vi "VP_RT_base.vi"() -> ()   [LabVIEW 2015] (continued)
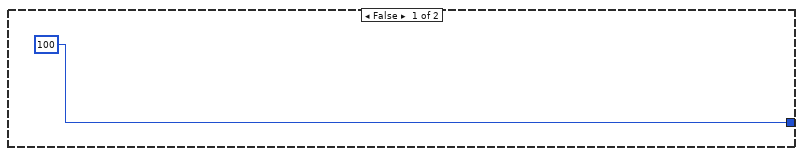
[diagram p2: hidden frame]
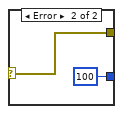
[diagram p3: hidden frame]
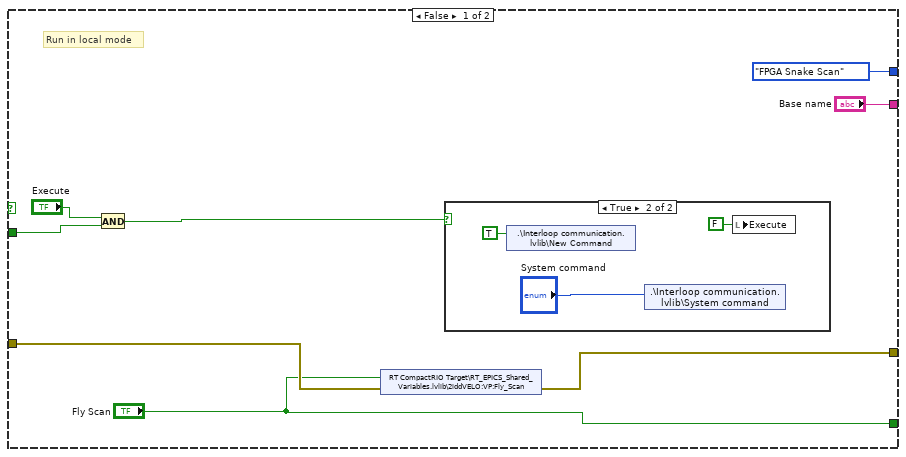
[diagram p4: hidden frame]
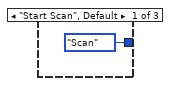
[diagram p7: hidden frame]
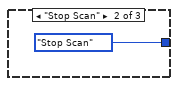
[diagram p8: hidden frame]
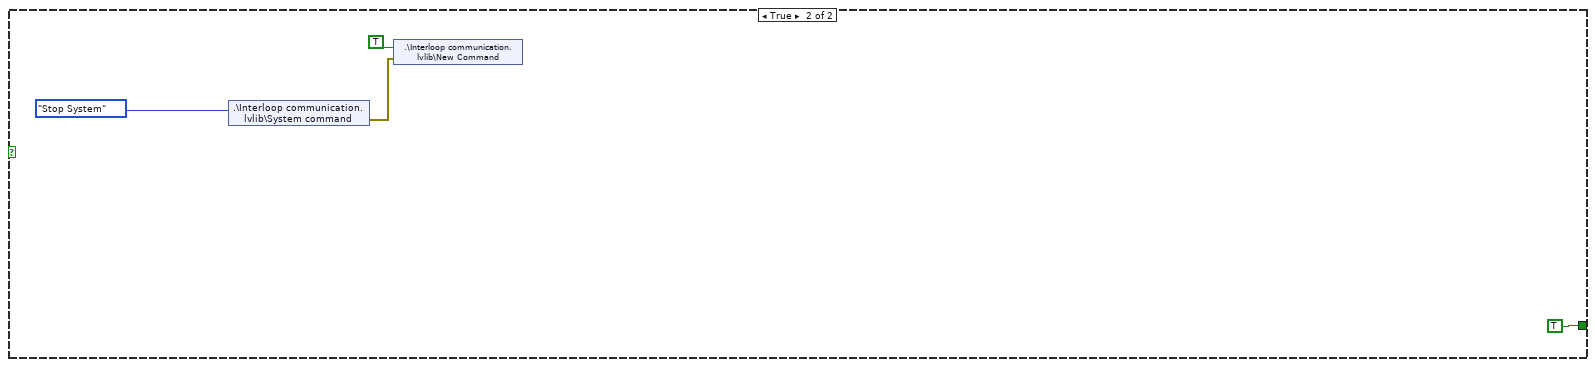
[diagram p9: hidden frame]
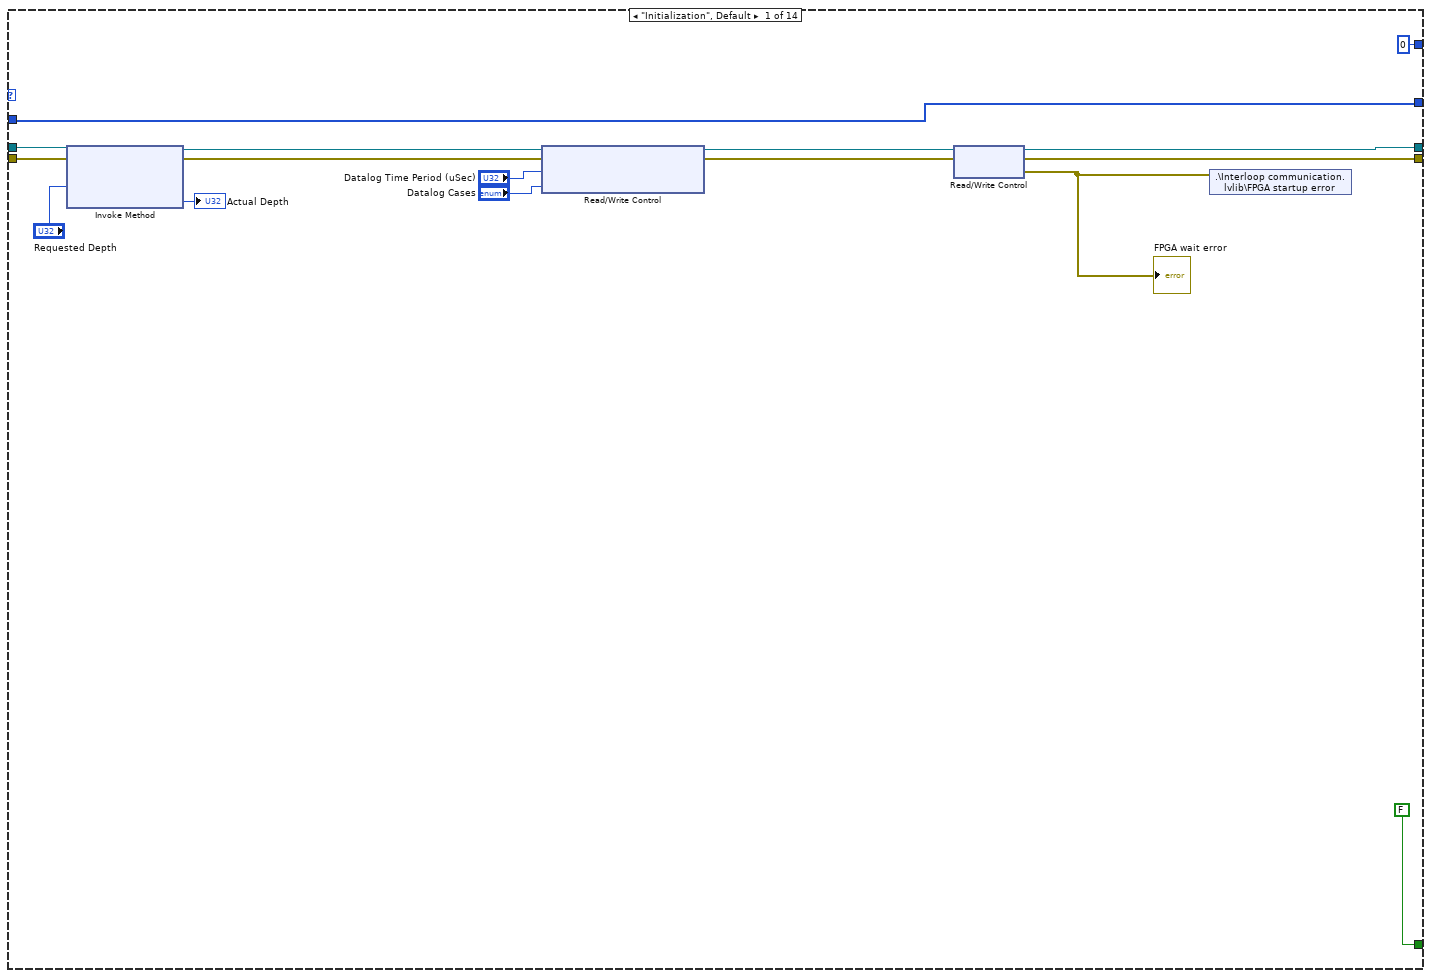
[diagram p10: hidden frame]
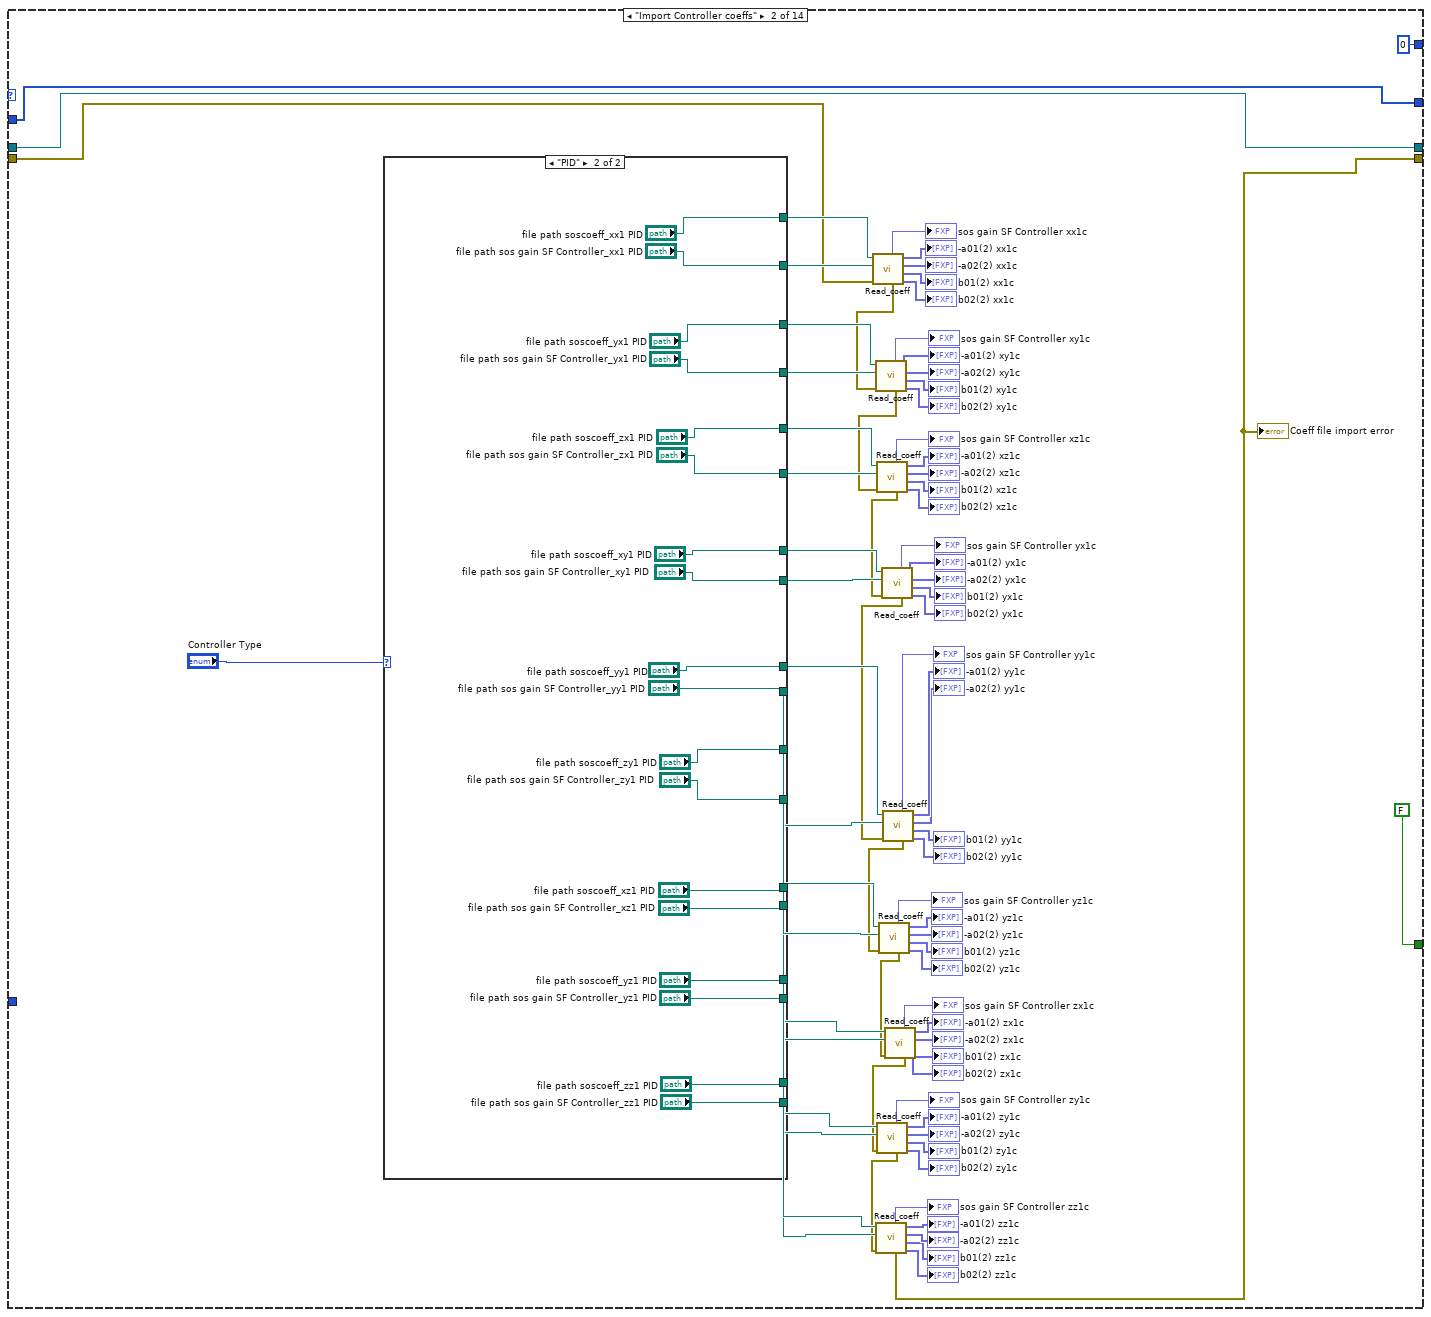
[diagram p11: hidden frame]
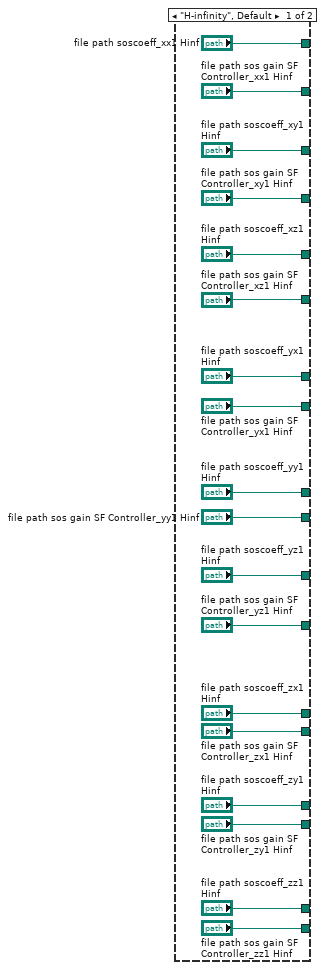
[diagram p12: hidden frame]
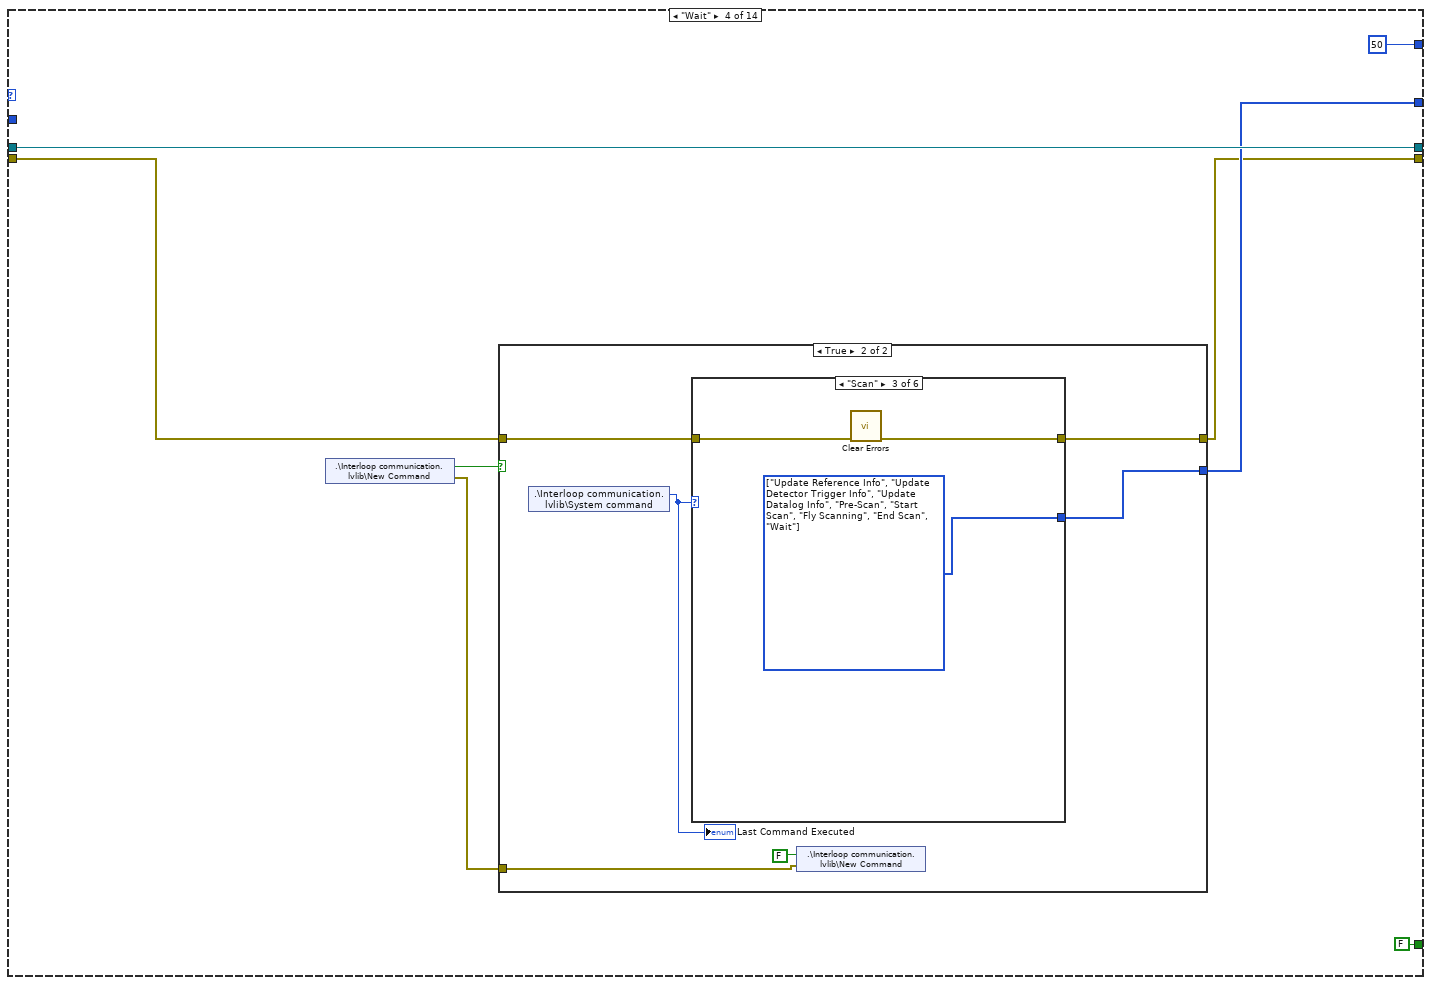
[diagram p13: hidden frame]
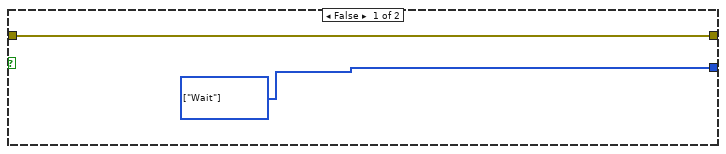
[diagram p14: hidden frame]
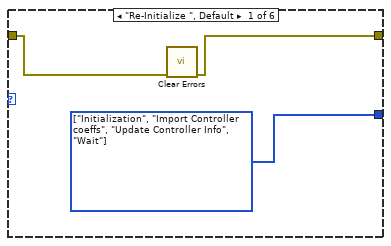
[diagram p15: hidden frame]
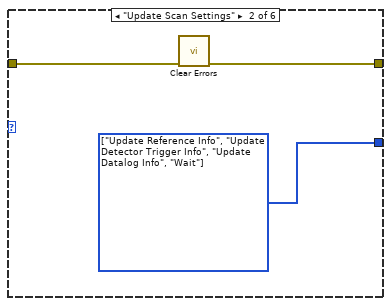
[diagram p16: hidden frame]
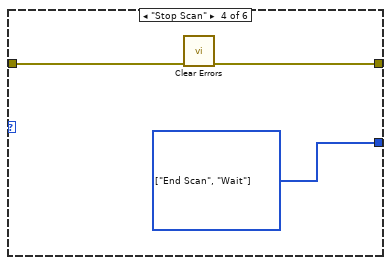
[diagram p17: hidden frame]
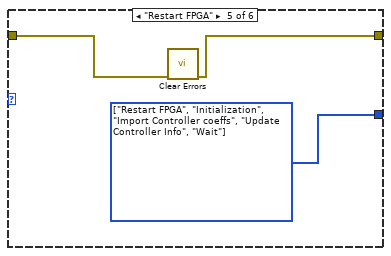
[diagram p18: hidden frame]
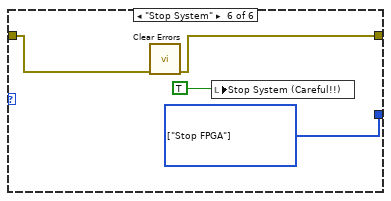
[diagram p19: hidden frame]
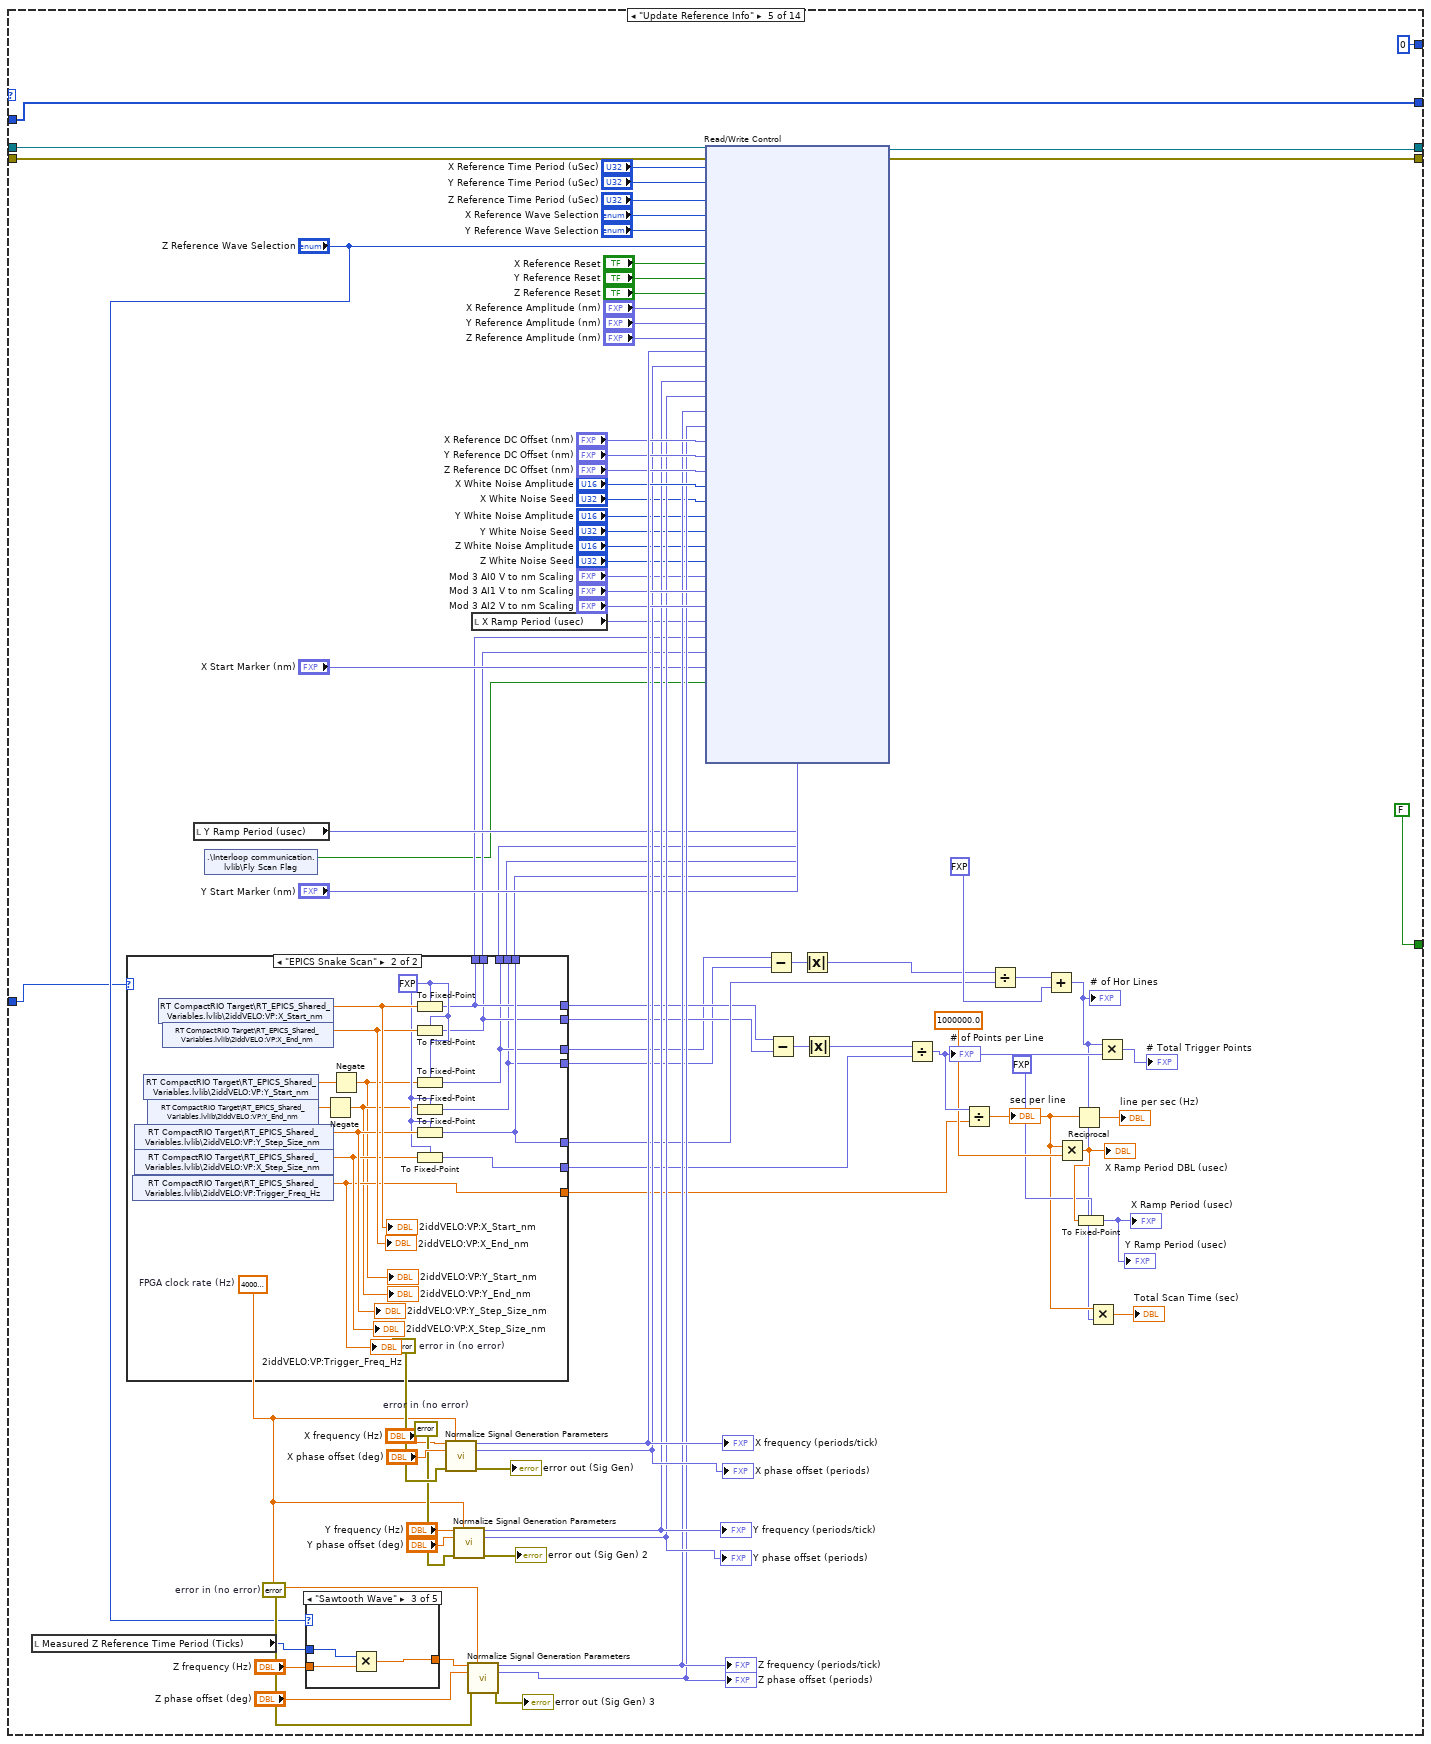
[diagram p20: hidden frame]
        n230 = case shown="False" w615 {
          tunnel: w614 -> [w668 w669]
          tunnel: [w666 w669] -> w613
          frame False {
            # "Either FIFO not empty or FPGA not \ndone running -- repeat scanning state"
            n231 = Insert Into Array(array=w668, index=0, new element=State_Enum."Fly Scanning" ("new element/subarray")) -> (w666:T11[])
          }
          frame True {
            # "FIFO empty, FPGA done running \n-- moving onto next state"
          }
        }
        n232 = Bundle("t0"=w662, w657, w658) -> (→"Reference and Actual positions":cluster{"t0":dbl, dbl, dbl[][]})  [unwired: 1 in]
        n233 = Array To Spreadsheet String(delimiter (Tab)=w634, array=w653, 3:w635) -> (spreadsheet string=w633:string)
        n234 = call "Convert to Dynamic Data"("Array"=w611) -> ("Dynamic Data Type"=w648:dynamicdata)  [unwired: 3 in]
        n235 = call "Convert to Dynamic Data2"("Array"=w610) -> ("Dynamic Data Type"=w642:dynamicdata)  [unwired: 3 in]
        n236 = call "Convert to Dynamic Data3"("Array"=w609) -> ("Dynamic Data Type"=w644:dynamicdata)  [unwired: 3 in]
        n237 = call "Convert to Dynamic Data4"("Array"=w608) -> ("Dynamic Data Type"=w643:dynamicdata)  [unwired: 3 in]
        n238 = call "Data_Write.vi"("error initialize"=w654, "Data"=w633, "Command List"=Data_Write_Control."Write") -> ("error out"=w632:errorcluster)  [unwired: 5 in, 1 out]
        n239 = To Double Precision Float(number=w611) -> (double precision float=w607:dbl[])
        n240 = To Double Precision Float(number=w610) -> (double precision float=w606:dbl[])
        n241 = To Double Precision Float(number=w609) -> (double precision float=w605:dbl[])
        n242 = To Double Precision Float(number=w608) -> (double precision float=w604:dbl[])
        n243 = call "Convert from Dynamic Data"("Dynamic Data Type"=w648) -> ("Array"=w649:dbl[])  [unwired: 3 in]
        n244 = call "Convert from Dynamic Data2"("Dynamic Data Type"=w642) -> ("Array"=w647:dbl[])  [unwired: 3 in]
        n245 = call "Convert from Dynamic Data3"("Dynamic Data Type"=w644) -> ("Array"=w646:dbl[])  [unwired: 3 in]
        n246 = call "Convert from Dynamic Data4"("Dynamic Data Type"=w643) -> ("Array"=w645:dbl[])  [unwired: 3 in]
        n247 = Bundle(w605, w604) -> (→"XY Graph 4":cluster{dbl[], dbl[]})  [unwired: 1 in]
        n248 = Bundle(w607, w606) -> (→"XY Graph 3":cluster{dbl[], dbl[]})  [unwired: 1 in]
        n249 = Bundle("Array"=w649, "Array"=w647) -> (→"XY Ref":cluster{"Array":dbl[], "Array":dbl[]})  [unwired: 1 in]
        n250 = Bundle("Array"=w646, "Array"=w645) -> (→"XY actual":cluster{"Array":dbl[], "Array":dbl[]})  [unwired: 1 in]
        n251 = Merge Errors(w638, w632) -> (w637:errorcluster)
      }
      frame "End Scan" {
        n252 = xnode "Invoke Method"("FPGA VI Reference In"=w675, "error in"=w673) -> ("FPGA VI Reference Out"=w674:refnum<k20>, "error out"=w672:errorcluster)
        n253 = xnode "Read/Write Control"("FPGA VI Reference In"=w674, "error in"=w672, "stop case"=TRUE ("New FPGA command")) -> ("FPGA VI Reference Out"=w678:refnum<k20>, "error out"=w677:errorcluster)
        n254 = shared-variable "RT CompactRIO Target\\RT_EPICS_Shared_Variables.lvlib\\2iddVELO:VP:Scanning"(FALSE ("2iddVELO:VP:Fly_Scanning")) -> ()  [unwired: 1 in, 1 out]
        n255 = call "Data_Write.vi"("error initialize"=w677, "Command List"=Data_Write_Control."Close") -> ("error out"=w671:errorcluster)  [unwired: 6 in, 1 out]
        n256 = case shown="No Error" w671 {
          tunnel: w671 -> [w689 w690]
          tunnel: [w688 w690] -> w681
          frame No Error {
            n257 = local read "Output filename"() -> (w685:string)
            n258 = local read "Output path"() -> (w686:path)
            n259 = Path To String(path=w686) -> (string=w684:string)
            n260 = shared-variable "RT CompactRIO Target\\RT_EPICS_Shared_Variables.lvlib\\2iddVELO:VP:Last_Filename"(w685, error in=w689) -> (error out=w687:errorcluster)
            n261 = shared-variable "RT CompactRIO Target\\RT_EPICS_Shared_Variables.lvlib\\2iddVELO:VP:cRIO_Dir"(w684, error in=w687) -> (error out=w688:errorcluster)
          }
          frame Error {
          }
        }
      }
      frame "Restart FPGA" {
        n262 = call <vilib>:"Clear Errors.vi"("error in (no error)"=w696) -> ("error out"=w697:errorcluster)  [unwired: 5 in, 1 out]
        n263 = xnode "Invoke Method"("FPGA VI Reference In"=w702, "error in"=w697) -> ("FPGA VI Reference Out"=w701:refnum<k20>, "error out"=w700:errorcluster)
        n264 = xnode "Read/Write Control"("FPGA VI Reference In"=w701, "error in"=w700, "stop case"=TRUE) -> ("FPGA VI Reference Out"=w695:refnum<k20>, "error out"=w694:errorcluster)
        n265 = xnode "Invoke Method"("FPGA VI Reference In"=w695, "error in"=w694) -> ("FPGA VI Reference Out"=w693:refnum<k20>, "error out"=w692:errorcluster)
      }
      frame "Stop FPGA" {
        w710 = T11[] [enum."Stop FPGA"] items=["Initialization", "Import Controller coeffs", "Update Controller Info", "Wait", "Update Reference Info", "Update Detector Trigger Info", "Update Datalog Info", "Check FPGA Status", "Pre-Scan", "Start Scan", "Step Scanning", "Fly Scanning", "End Scan", "Restart FPGA", "Stop FPGA"] ("Reduced Array of States")
        w709 = TRUE ("stop case")
        n266 = xnode "Invoke Method"("FPGA VI Reference In"=w717, "error in"=w716) -> ("FPGA VI Reference Out"=w715:refnum<k20>, "error out"=w714:errorcluster)
        n267 = xnode "Read/Write Control"("FPGA VI Reference In"=w715, "error in"=w714, "stop case"=w709, "New FPGA command"=w709, "FPGA command"=enum16{"Start Scan", "Shutdown"}."Shutdown") -> ("FPGA VI Reference Out"=w713:refnum<k20>, "error out"=w706:errorcluster)
        n268 = xnode "Invoke Method"("FPGA VI Reference In"=w713, "error in"=w706) -> ("FPGA VI Reference Out"=w707:refnum<k20>, "error out"=w705:errorcluster)
        n269 = xnode "Close FPGA VI Reference"("FPGA VI Reference In"=w707, "error in"=w705) -> ("error out"=w712:errorcluster)
      }
    }
    "Main Loop error" <- w105
    n270 = shared-variable ".\\Interloop communication.lvlib\\Main Loop Error"(w105) -> ()  [unwired: 1 in, 1 out]
    n271 = node-c288(w100) -> ()  [unwired: 1 out]
    n272 = call "State Control.vi"("Stop"=FALSE, "Array of States"=w107, "Error Input"=w105) -> ("Next State"=w97:T11, "Reduced Array of States"=w101:T11[])  [unwired: 5 in]
    "RT Main Loop State" <- w94
    "Main Loop Iterations" <- w103
    "Reduced Array of States" <- w102
  }
  n273 = while {
    tunnel: w2 -> [w726]
    tunnel: w1 -> [w725]
    i -> [w723]
    stop <- w724 stop-if-true
    # "Readback loop"
    n274 = local read "RT Main Loop State"() -> (w729:T11)
    n275 = Not Equal?(x=w729, y=State_Enum."Initialization") -> (x != y?=w727:bool)
    n276 = case shown="True" w727 {
      tunnel: w726 -> [_ w737]
      tunnel: w725 -> [_ w735]
      tunnel: [u32 100 ("milliseconds to wait") "Readback Loop time between iterations (ms)"] -> w722
      frame False {
      }
      frame True {
        w776 = 40000000.0  # FPGA Clock Rate (Hz)
        w795 = 40000000.0  # FPGA Clock Rate (Hz)
        w812 = 40000000.0  # FPGA Clock Rate (Hz)
        n277 = xnode "Read/Write Control"("FPGA VI Reference In"=w737, "error in"=w735) -> ("FPGA VI Reference Out"=w736:refnum<k20>, "error out"=w734:errorcluster, "FPGA state"=w733:T10, "Fly scan completed"=→"Fly Scan Complete":bool)
        "FPGA state" <- w733
        n278 = Format Into String(format string="%s", w733) -> (resulting string=w732:string)  [unwired: 2 in, 1 out]
        n279 = xnode "Read/Write Control"("FPGA VI Reference In"=w736, "error in"=w734) -> ("error out"=w743:errorcluster, "Measured Datalog Time Period (Ticks)"=w770:u32, "Measured Counter Time Period (Ticks)"=w775:u32, "Mod4/DIO0"=→"Mod4/DIO0":bool, "Mod4/DIO1"=→"Mod4/DIO1":bool, "Mod4/DIO2"=→"Mod4/DIO2":bool, "Mod4/DIO3"=→"Mod4/DIO3":bool, "Mod5/DIO0"=→"Mod5/DIO0":bool, "Mod5/DIO1"=→"Mod5/DIO1":bool, "Mod5/DIO2"=→"Mod5/DIO2":bool, "Mod5/DIO3"=→"Mod5/DIO3":bool, "Mod6/DIO0"=→"Mod6/DIO0":bool, "Mod6/DIO1"=→"Mod6/DIO1":bool, "Mod6/DIO2"=→"Mod6/DIO2":bool, "Mod6/DIO3"=→"Mod6/DIO3":bool, "32 bit Count Optics X"=→"32 bit Count Optics X":i32, "32 bit Count Optics  Y"=→"32 bit Count Optics  Y":i32, "32 bit Count Optics  Z"=→"32 bit Count Optics  Z":i32, "32 bit Count Sample X"=→"32 bit Count Sample X":i32, "32 bit Count Sample  Y"=→"32 bit Count Sample  Y":i32, "32 bit Count Sample  Z"=→"32 bit Count Sample  Z":i32, "Optics X Stage Displacement (nm)"=→"Optics X Stage Displacement (nm)":fxp<+/-,58,25>, "Optics Y Stage Displacement (nm)"=→"Optics Y Stage Displacement (nm)":fxp<+/-,58,25>, "Optics Z Stage Displacement (nm)"=→"Optics Z Stage Displacement (nm)":fxp<+/-,58,25>, "Sample X Stage Displacement (nm)"=→"Sample X Stage Displacement (nm)":fxp<+/-,58,25>, "Sample Y Stage Displacement (nm)"=→"Sample Y Stage Displacement (nm)":fxp<+/-,58,25>, "Sample Z Stage Displacement (nm)"=→"Sample Z Stage Displacement (nm)":fxp<+/-,58,25>)  [unwired: 1 out]
        "Measured Datalog Time Period (Ticks)" <- w770
        "Measured Counter Time Period (Ticks)" <- w775
        n280 = xnode "Read/Write Control"("FPGA VI Reference In"=w736, "error in"=w734) -> ("error out"=w742:errorcluster, "Measured Detector Trigger Time Period (Ticks)"=→"Measured Detector Trigger Time Period (Ticks)":u32, "Measured Trigger Gen Time Period (Ticks)"=→"Measured Trigger Gen Time Period (Ticks)":u32, "Detector Trigger (V)"=→"Detector Trigger (V)":fxp<+/-,20,5>, "Detector Trigger In Range?"=→"Detector Trigger In Range?":bool, "Measured Data Trigger Time Period (Ticks)"=→"Measured Data Trigger Time Period (Ticks)":u32, "Trigger for Data"=→"Trigger for Data":fxp<+/-,58,25>)  [unwired: 1 out]
        n281 = xnode "Read/Write Control"("FPGA VI Reference In"=w736, "error in"=w734) -> ("error out"=w740:errorcluster, "PI X-Stage Input (V)"=→"PI X-Stage Input (V)":fxp<+/-,20,5>, "PI Y-Stage Input (V)"=→"PI Y-Stage Input (V)":fxp<+/-,20,5>, "PI Z-Stage Input (V)"=→"PI Z-Stage Input (V)":fxp<+/-,20,5>, "X-Stage Input In Range?"=→"X-Stage Input In Range?":bool, "Y-Stage Input In Range?"=→"Y-Stage Input In Range?":bool, "Z-Stage Input In Range?"=→"Z-Stage Input In Range?":bool, "Measured Controller Time Period (Ticks)"=w816:u32, "Measured Controller Output Time Period (Ticks)"=w815:u32, "Measured Plant Output Time Period (Ticks)"=w814:u32, "Measured Analog Input Time Period (Ticks)"=w813:u32)  [unwired: 1 out]
        "Measured Controller Time Period (Ticks)" <- w816
        "Measured Controller Output Time Period (Ticks)" <- w815
        "Measured Plant Output Time Period (Ticks)" <- w814
        "Measured Analog Input Time Period (Ticks)" <- w813
        n282 = xnode "Read/Write Control"("FPGA VI Reference In"=w736, "error in"=w734) -> ("error out"=w741:errorcluster, "X Stage Reference (nm)"=→"X Stage Reference (nm)":fxp<+/-,58,25>, "Y Stage Reference (nm)"=→"Y Stage Reference (nm)":fxp<+/-,58,25>, "Z Stage Reference (nm)"=→"Z Stage Reference (nm)":fxp<+/-,58,25>, "Measured X Reference Time Period (Ticks)"=w797:u32, "Measured Y Reference Time Period (Ticks)"=w796:u32, "Measured Z Reference Time Period (Ticks)"=w788:u32, "Fly Scan Running"=→"Fly Scan Running":bool, "Continue Run"=→"Continue Run":bool)  [unwired: 1 out]
        "Measured X Reference Time Period (Ticks)" <- w797
        "Measured Y Reference Time Period (Ticks)" <- w796
        "Measured Z Reference Time Period (Ticks)" <- w788
        n283 = shared-variable "RT CompactRIO Target\\RT_EPICS_Shared_Variables.lvlib\\2iddVELO:VP:FPGA_State"(w732) -> ()  [unwired: 1 in, 1 out]
        n284 = call "Convert Measured Rate.vi"("FPGA Clock Rate (Hz)"=w795, "Measured Reference Time Period (Ticks)"=w788) -> ("Measured Reference Loop Rate (kHz)"=→"Measured Z Reference Loop Rate (kHz)":dbl, "Measured Reference Loop Period (s)"=→"Measured Z Reference Loop Rate (secs)":dbl)
        n285 = call "Convert Measured Rate.vi"("FPGA Clock Rate (Hz)"=w795, "Measured Reference Time Period (Ticks)"=w796) -> ("Measured Reference Loop Rate (kHz)"=→"Measured Y Reference Loop Rate (kHz)":dbl, "Measured Reference Loop Period (s)"=→"Measured Y Reference Loop Rate (secs)":dbl)
        n286 = call "Convert Measured Rate.vi"("FPGA Clock Rate (Hz)"=w776, "Measured Reference Time Period (Ticks)"=w775) -> ("Measured Reference Loop Rate (kHz)"=w773:dbl, "Measured Reference Loop Period (s)"=→"Measured Counter Loop Rate (secs)":dbl)
        n287 = call "Convert Measured Rate.vi"("FPGA Clock Rate (Hz)"=w795, "Measured Reference Time Period (Ticks)"=w797) -> ("Measured Reference Loop Rate (kHz)"=→"Measured X Reference Loop Rate (kHz)":dbl, "Measured Reference Loop Period (s)"=→"Measured X Reference Loop Rate (secs)":dbl)
        n288 = call "Convert Measured Rate.vi"("FPGA Clock Rate (Hz)"=w776, "Measured Reference Time Period (Ticks)"=w770) -> ("Measured Reference Loop Rate (kHz)"=→"Measured Datalog Loop Rate (kHz)":dbl, "Measured Reference Loop Period (s)"=→"Measured Datalog Loop Rate (secs)":dbl)
        n289 = call "Convert Measured Rate.vi"("FPGA Clock Rate (Hz)"=w812, "Measured Reference Time Period (Ticks)"=w816) -> ("Measured Reference Loop Rate (kHz)"=→"Measured Controller Loop Rate (kHz)":dbl, "Measured Reference Loop Period (s)"=→"Measured Controller Loop Rate (secs)":dbl)
        n290 = call "Convert Measured Rate.vi"("FPGA Clock Rate (Hz)"=w812, "Measured Reference Time Period (Ticks)"=w815) -> ("Measured Reference Loop Rate (kHz)"=→"Measured Controller Output Loop Rate (kHz)":dbl, "Measured Reference Loop Period (s)"=→"Measured Controller Output Loop Rate (secs)":dbl)
        n291 = call "Convert Measured Rate.vi"("FPGA Clock Rate (Hz)"=w812, "Measured Reference Time Period (Ticks)"=w814) -> ("Measured Reference Loop Rate (kHz)"=→"Measured Plant Output Loop Rate (kHz)":dbl, "Measured Reference Loop Period (s)"=→"Measured Plant Output Loop Rate (secs)":dbl)
        n292 = call "Convert Measured Rate.vi"("FPGA Clock Rate (Hz)"=w812, "Measured Reference Time Period (Ticks)"=w813) -> ("Measured Reference Loop Rate (kHz)"=→"Measured Analog Input Loop Rate (kHz)":dbl, "Measured Reference Loop Period (s)"=→"Measured Analog Input Loop Rate (secs)":dbl)
        n293 = Divide(x=w773, y=1000.0) -> (x/y=→"Measured Counter Loop Rate (MHz)":dbl)
        n294 = Merge Errors(w740, w741, w742, w743) -> (w739:errorcluster)
        "Readback error" <- w739
        n295 = shared-variable ".\\Interloop communication.lvlib\\Readback Loop Error"(w739) -> ()  [unwired: 1 in, 1 out]
      }
    }
    n296 = local read "Stop System (Careful!!)"() -> (w724:bool)
    n297 = Wait (ms)(milliseconds to wait=w722) -> ()  [unwired: 1 out]
    "Readback loop Iterations" <- w723
  }
  n298 = while {
    stop <- w834 stop-if-true
    n299 = shared-variable "RT CompactRIO Target\\RT_EPICS_Shared_Variables.lvlib\\2iddVELO:VP:Scan_Type"() -> (w820:string, error out=w819:errorcluster)  [unwired: 1 in]
    "2iddVELO:VP:Scan_Type" <- w820
    n300 = shared-variable "RT CompactRIO Target\\RT_EPICS_Shared_Variables.lvlib\\2iddVELO:VP:Controller_Type"() -> (w827:string, error out=w828:errorcluster)  [unwired: 1 in]
    "2iddVELO:VP:Controller_Type" <- w827
    n301 = shared-variable "RT CompactRIO Target\\RT_EPICS_Shared_Variables.lvlib\\2iddVELO:VP:cRIO_Command"() -> (w826:string, error out=w825:errorcluster)  [unwired: 1 in]
    "2iddVELO:VP:cRIO_Command" <- w826
    n302 = Scan From String(input string=w820, error in=w819, default 1=Scan_type."Fly" ("Scan type")) -> (error out=w818:errorcluster, output 1=→"EPICS Scan Type":T13)  [unwired: 2 in, 2 out]
    n303 = Scan From String(input string=w826, error in=w825, default 1=EPICS_Command_Control."Start Scan" ("default value 1")) -> (error out=w824:errorcluster, output 1=→"EPICS cRIO Command":T12)  [unwired: 2 in, 2 out]
    n304 = Scan From String(input string=w827, error in=w828, default 1=Controller_Type."H-infinity" ("Controller Type")) -> (error out=w823:errorcluster, output 1=→"EPICS Controller Type":T2)  [unwired: 2 in, 2 out]
    n305 = Merge Errors(w824, w823, w818) -> (w833:errorcluster)
    "EPICS command error" <- w833
    n306 = local read "Stop System (Careful!!)"() -> (w834:bool)
    n307 = shared-variable ".\\Interloop communication.lvlib\\EPICS command error"(w833) -> ()  [unwired: 1 in, 1 out]
    n308 = Wait Until Next ms Multiple(millisecond multiple=u32 100) -> ()  [unwired: 1 out]
  }
  n309 = node-c288(w8) -> (→"Timed Loop (end error)":errorcluster, →"Iteration Duration RT Timed-Loop":i64)
